vi "UHR-Fleezers Control (host) - 12.7.vi"() -> ()   [LabVIEW 2012] (continued)
              }
              frame True {
                n386 = stacked-sequence {
                  tunnel: w654 -> [_ _ _ _ _ _ _ _ _ w675 _ _]
                  tunnel: w653 -> [_ _ _ _ _ _ _ _ _ w673 _ _]
                  frame #0 {
                    n387 = property on="Save ave N" class="DigNum (strict)"("Val(Sgnl)"=1.0 ("Value (Signaling)")) -> ()  [unwired: 2 in, 2 out]
                  }
                  frame #1 {
                    n388 = Wait (ms)(milliseconds to wait=u32 500) -> ()  [unwired: 1 out]
                  }
                  frame #2 {
                    n389 = property on="Trap Delta (MHz)" class="DigNum (strict)"("Val(Sgnl)"="Offset 2 Start (MHz)") -> ()  [unwired: 2 in, 2 out]
                    n390 = Replace Array Subset(array=u32[] [0] ("Index Values"), new element="Offset 2 Set", index=0) -> (w659:u32[])
                    n391 = property on="Saved AOD Raster Scan Parameter Sets" class="Arr (strict)"("Index Values"=w659) -> ()  [unwired: 2 in, 2 out]
                  }
                  frame #3 {
                    n392 = Wait (ms)(milliseconds to wait=u32 500) -> ()  [unwired: 1 out]
                  }
                  frame #4 {
                    n393 = property on="Load parameters" class="Bool (strict)"("Val(Sgnl)"=TRUE ("Value (Signaling)")) -> ()  [unwired: 2 in, 2 out]
                  }
                  frame #5 {
                    n394 = Wait (ms)(milliseconds to wait=u32 500) -> ()  [unwired: 1 out]
                  }
                  frame #6 {
                    n395 = property on="Trap Raster Scan" class="Bool (strict)"("Val(Sgnl)"=TRUE ("Value (Signaling)")) -> ()  [unwired: 2 in, 2 out]
                  }
                  frame #7 {
                    n396 = Wait (ms)(milliseconds to wait=u32 2000) -> ()  [unwired: 1 out]
                  }
                  frame #8 {
                    n397 = while {
                      stop <- w668 stop-if-true
                      n398 = local read "Raster Scanning..."() -> (w671:bool)
                      n399 = local read "Saving..."() -> (w669:bool)
                      n400 = Wait (ms)(milliseconds to wait=u32 100) -> ()  [unwired: 1 out]
                      n401 = Not(x=w669) -> (.not. x?=w667:bool)
                      n402 = Not(x=w671) -> (.not. x?=w670:bool)
                      n403 = And(x=w670, y=w667) -> (x .and. y?=w668:bool)
                    }
                  }
                  frame #9 {
                    n404 = property on="Trap Delta (MHz)" class="DigNum (strict)"("Val(Sgnl)"=w675) -> ()  [unwired: 2 in, 2 out]
                    n405 = property on="Saved AOD Raster Scan Parameter Sets" class="Arr (strict)"("Index Values"=u32[] [0]) -> ()  [unwired: 2 in, 2 out]
                    n406 = property on="Save ave N" class="DigNum (strict)"("Val(Sgnl)"=w673) -> ()  [unwired: 2 in, 2 out]
                  }
                  frame #10 {
                    n407 = Wait (ms)(milliseconds to wait=u32 500) -> ()  [unwired: 1 out]
                  }
                  frame #11 {
                    n408 = property on="Load parameters" class="Bool (strict)"("Val(Sgnl)"=TRUE ("Value (Signaling)")) -> ()  [unwired: 2 in, 2 out]
                  }
                }
              }
            }
          }
          frame #9 {
            n409 = property on="Read Cal" class="Bool (strict)"("Val(Sgnl)"=TRUE ("Value (Signaling)")) -> ()  [unwired: 2 in, 2 out]
          }
          frame #10 {
            n410 = Wait (ms)(milliseconds to wait=u32 1000) -> ()  [unwired: 1 out]
          }
          frame #11 {
            n411 = property on="Fish for Tether" class="Bool (strict)"("Val(Sgnl)"=TRUE ("Value (Signaling)")) -> ()  [unwired: 2 in, 2 out]
          }
        }
        n412 = local write "Cal/Data Acq. Spot"(FALSE ("Cal/Data Acq. Spot")) -> ()
      }
      event "Dump Beads": Value Change {
        n413 = event-data() -> ()  [unwired: 1 in, 5 out]
        n414 = flat-sequence {
          tunnel: ["Dump spot flow on?"] -> w681
          tunnel: [w692] -> w682
          tunnel: w681 -> [w692]
          tunnel: w685 -> [w697]
          tunnel: w684 -> [w696]
          tunnel: [w694] -> w683
          tunnel: w682 -> [w694]
          tunnel: w683 -> [w707]
          frame #0 {
            w686 = FALSE ("Value (Signaling)")
            n415 = local read "Saving..."() -> (w688:bool)
            n416 = local write "Dump Beads"(FALSE ("Dump Beads")) -> ()
            n417 = property on="Inject Pump 3" class="Bool (strict)"("Val(Sgnl)"=w686) -> ()  [unwired: 2 in, 2 out]
            n418 = property on="Inject Pump 1" class="Bool (strict)"("Val(Sgnl)"=w686) -> ()  [unwired: 2 in, 2 out]
            n419 = local write "Stop Saving"(w688) -> ()
          }
          frame #1 {
            w689 = FALSE ("Fl. Triggered...")
            n420 = case shown="True" "Dump spot flow on?" {
              frame False {
              }
              frame True {
                n421 = property on="Sample Channel\nFlow" class="Bool (strict)"("Val(Sgnl)"=TRUE ("Stage Moving")) -> ()  [unwired: 2 in, 2 out]
              }
            }
            n422 = local write "Fl. Triggered..."(w689) -> ()
            n423 = local write "Tether"(w689) -> ()
            n424 = property on="Green Laser ON" class="Bool (strict)"("Val(Sgnl)"=w689) -> ()  [unwired: 2 in, 2 out]
            n425 = property on="Trap Pos. FB ON" class="Bool (strict)"("Val(Sgnl)"=w689) -> ()  [unwired: 2 in, 2 out]
            n426 = property on="Trap Trig. Fl." class="Bool (strict)"("Val(Sgnl)"=w689) -> ()  [unwired: 2 in, 2 out]
            n427 = property on="Fl. Triggered..." class="Bool (strict)"("Val(Sgnl)"=w689) -> ()  [unwired: 2 in, 2 out]
            n428 = property on="Dip for Protein" class="Bool (strict)"("Val(Sgnl)"=w689) -> ()  [unwired: 2 in, 2 out]
            n429 = property on="Pause dwell" class="Bool (strict)"("Val(Sgnl)"=w689) -> ()  [unwired: 2 in, 2 out]
          }
          frame #2 {
            n430 = property on="Trap Pos. FB Offset Factor" class="DigNum (strict)"("Val(Sgnl)"=i64 0 ("Value (Signaling)")) -> ()  [unwired: 2 in, 2 out]
          }
          frame #3 {
            n431 = local read "Saved Stage Positions"() -> (w698:dbl[][])
            n432 = local write "Stage Moving"(TRUE ("Stage Moving")) -> ()
            n433 = Array Subset(array=w698, index (row)=3 ("index"), length (row)=1 ("length"), index (col)=1 ("index"), length (col)=3 ("length")) -> (w703:dbl[][])
            n434 = Reshape Array(w703, 3 ("dimension size")) -> (w701:dbl[])
            n435 = Array To Cluster(array=w701) -> (cluster=w700:cluster{"[0]":dbl, "[1]":dbl, "[2]":dbl})
            n436 = call "Set Stage Position.vi"("Position"=w700, "error in"=w696, "VISA resource name in"=w697) -> ()  [unwired: 3 out]
          }
          frame #4 {
            w708 = FALSE ("Value (Signaling)")
            n437 = case shown="True" w707 {
              frame False {
              }
              frame True {
                n438 = property on="Sample Channel\nFlow" class="Bool (strict)"("Val(Sgnl)"=FALSE ("Stage Moving")) -> ()  [unwired: 2 in, 2 out]
              }
            }
            n439 = property on="Trap 1 (ON/OFF)" class="Bool (strict)"("Val(Sgnl)"=w708) -> ()  [unwired: 2 in, 2 out]
            n440 = property on="Trap 2 (ON/OFF)" class="Bool (strict)"("Val(Sgnl)"=w708) -> ()  [unwired: 2 in, 2 out]
            n441 = call <vilib>:"Beep.vi"() -> ()  [unwired: 3 in, 9 out]
          }
          frame #5 {
            n442 = property on="Move Cap. 2 (ADig Top)" class="Bool (strict)"("Val(Sgnl)"=TRUE ("Value (Signaling)")) -> ()  [unwired: 2 in, 2 out]
            n443 = property on="Tab Control" class="TabCtl (strict)"("Val(Sgnl)"=T26."Status" ("Value (Signaling)")) -> ()  [unwired: 2 in, 2 out]
          }
        }
      }
      event "Dip for Protein": Value Change {
        n444 = event-data() -> ()  [unwired: 1 in, 5 out]
        n445 = case shown="True" "Dip for Protein" {
          tunnel: w714 -> [_ w716]
          tunnel: w713 -> [_ w715]
          frame False {
          }
          frame True {
            n446 = while {
              tunnel: w716 -> [w727]
              tunnel: w715 -> [w726]
              i -> [w721]
              stop <- w723 stop-if-true
              n447 = Increment(x=w721) -> (x+1=→"Dip #":i32)
              n448 = flat-sequence {
                tunnel: w726 -> [w738]
                tunnel: w727 -> [w739]
                tunnel: [w739] -> w731
                tunnel: [w738] -> w730
                tunnel: [w732] -> w717
                tunnel: [w744] -> w725
                tunnel: [w745] -> w724
                tunnel: w731 -> [w746]
                tunnel: w730 -> [w747]
                tunnel: [w742] -> w718
                tunnel: w717 -> [w742]
                tunnel: [w755] -> w729
                tunnel: w725 -> [w755]
                tunnel: [w754] -> w728
                tunnel: w724 -> [w754]
                tunnel: [w751] -> w722
                tunnel: [w750] -> w719
                tunnel: w718 -> [w750]
                tunnel: w728 -> [w775]
                tunnel: w729 -> [w776]
                tunnel: w722 -> [w777]
                tunnel: w719 -> [w774]
                tunnel: [w833] -> w723
                frame #0 {
                  n449 = local read "Trap Pos. FB ON"() -> (w732:bool)
                  n450 = Compound Arithmetic op=AND("Flow ON\nduring dip?", "FB OFF when \nflow ON", w732) -> (w733:bool)
                  n451 = case shown="True" "Move trap \nbefore dip move?" {
                    frame False {
                    }
                    frame True {
                      n452 = property on="Trap Delta (MHz)" class="DigNum (strict)"("Val(Sgnl)"="Dipping Delta (MHz)") -> ()  [unwired: 2 in, 2 out]
                    }
                  }
                  n453 = property on="Green Laser ON" class="Bool (strict)"("Val(Sgnl)"="Green ON\nbefore dip?") -> ()  [unwired: 2 in, 2 out]
                  n454 = property on="Sample Channel\nFlow" class="Bool (strict)"("Val(Sgnl)"="Flow ON\nduring dip?") -> ()  [unwired: 2 in, 2 out]
                  n455 = case shown="True" w733 {
                    frame False {
                    }
                    frame True {
                      n456 = property on="Trap Pos. FB ON" class="Bool (strict)"("Val(Sgnl)"=FALSE ("Value (Signaling)")) -> ()  [unwired: 2 in, 2 out]
                    }
                  }
                }
                frame #1 {
                  n457 = local read "Saved Stage Positions"() -> (w749:dbl[][])
                  n458 = local write "Cancel dwell"(FALSE ("Cancel dwell")) -> ()
                  n459 = call "move to saved stage position.vi"("error in"=w747, "Stage VISA resource name in"=w746, "Position"="Dip Stage \nPosition", "Saved Stage Positions"=w749) -> ("VISA resource name out"=w744:refnum<visa-resource-name>, "error out"=w745:errorcluster)
                }
                frame #2 {
                  n460 = node-c288() -> (w753:T23)  [unwired: 4 in]
                  n461 = timed-loop {
                    timing: w753 -> [_]
                    timing-out: [_] -> w752
                    tunnel: [w759] -> w751
                    i -> [w756]
                    stop <- w760 stop-if-true
                    n462 = node-c288() -> ()  [unwired: 1 in, 1 out]
                    n463 = Greater Or Equal?(x=w756, y="Dip Duration (s)") -> (x >= y?=w768:bool)
                    n464 = local read "Dip for Protein"() -> (w761:bool)
                    n465 = local read "Dump Beads"() -> (w758:bool)
                    n466 = local read "Cancel dwell"() -> (w767:bool)
                    n467 = local read "Pause dwell"() -> (w764:bool)
                    n468 = Not(x=w761) -> (.not. x?=w766:bool)
                    n469 = Compound Arithmetic op=OR(w767, w768, w766) -> (w765:bool)
                    n470 = Select(t=FALSE, s=w764, f=w765) -> (s? t:f=w762:bool)
                    n471 = Not(x=w758) -> (.not. x?=w757:bool)
                    n472 = node-c288() -> ()  [unwired: 1 in, 1 out]
                    n473 = And(x=w761, y=w757) -> (x .and. y?=w759:bool)
                    n474 = Or(x=w762, y=w758) -> (x .or. y?=w760:bool)
                    "Dip Time (s)" <- w756
                  }
                  n475 = node-c288(w752) -> ()  [unwired: 1 out]
                }
                frame #3 {
                  n476 = case shown="True" w777 {
                    tunnel: w776 -> [_ w782]
                    tunnel: w775 -> [_ w781]
                    tunnel: w774 -> [_ w778]
                    frame False {
                    }
                    frame True {
                      n477 = flat-sequence {
                        tunnel: w781 -> [w786]
                        tunnel: w782 -> [w787]
                        tunnel: [w787] -> w780
                        tunnel: [w786] -> w779
                        tunnel: w778 -> [w783]
                        tunnel: w780 -> [w797]
                        tunnel: w779 -> [w796]
                        tunnel: w778 -> [w805]
                        frame #0 {
                          n478 = local read "Sample Channel\nFlow"() -> (w785:bool)
                          n479 = case shown="True" w785 {
                            tunnel: "Flow ON \nduring return\nfrom dip?" -> [w788 w791]
                            tunnel: w783 -> [_ w790]
                            frame False {
                              n480 = case shown="True" w788 {
                                frame False {
                                }
                                frame True {
                                n481 = property on="Sample Channel\nFlow" class="Bool (strict)"("Val(Sgnl)"=TRUE ("Value (Signaling)")) -> ()  [unwired: 2 in, 2 out]
                                }
                              }
                            }
                            frame True {
                              n482 = case shown="False" w791 {
                                tunnel: w790 -> [w792 _]
                                frame False {
                                n483 = property on="Trap Pos. FB ON" class="Bool (strict)"("Val(Sgnl)"=w792) -> ()  [unwired: 2 in, 2 out]
                                n484 = property on="Sample Channel\nFlow" class="Bool (strict)"("Val(Sgnl)"=FALSE ("Value (Signaling)")) -> ()  [unwired: 2 in, 2 out]
                                }
                                frame True {
                                }
                              }
                            }
                          }
                        }
                        frame #1 {
                          # "For turning on green laser before stage reaches lower spot"
                          n485 = case shown="True" "Green ON\nafter start\nreturn?" {
                            frame False {
                            }
                            frame True {
                              n486 = flat-sequence {
                                frame #0 {
                                n487 = Multiply(x="Green delay after \nstart return (s)", y=1000.0) -> (x*y=w802:dbl)
                                n488 = Wait (ms)(milliseconds to wait=w802) -> ()  [unwired: 1 out]
                                }
                                frame #1 {
                                n489 = property on="Green Laser ON" class="Bool (strict)"("Val(Sgnl)"=TRUE ("Value (Signaling)")) -> ()  [unwired: 2 in, 2 out]
                                }
                              }
                            }
                          }
                          n490 = local read "Saved Stage Positions"() -> (w800:dbl[][])
                          n491 = local write "Cancel dwell"(FALSE ("Cancel dwell")) -> ()
                          n492 = call "move to saved stage position.vi"("error in"=w796, "Stage VISA resource name in"=w797, "Position"="Return Stage \nPosition", "Saved Stage Positions"=w800) -> ("error out"=w798:errorcluster)  [unwired: 1 out]
                          n493 = local write "Stage Control Serial Error"(w798) -> ()
                        }
                        frame #2 {
                          n494 = property on="Trap Pos. FB ON" class="Bool (strict)"("Val(Sgnl)"=w805) -> ()  [unwired: 2 in, 2 out]
                          n495 = case shown="True" "Green ON \nafter return?" {
                            frame False {
                            }
                            frame True {
                              n496 = property on="Green Laser ON" class="Bool (strict)"("Val(Sgnl)"=TRUE ("Value (Signaling)")) -> ()  [unwired: 2 in, 2 out]
                            }
                          }
                          n497 = case shown="True" "Move trap after return?" {
                            frame False {
                            }
                            frame True {
                              n498 = property on="Trap Delta (MHz)" class="DigNum (strict)"("Val(Sgnl)"="Dip Trap Delta 2 (MHz)") -> ()  [unwired: 2 in, 2 out]
                            }
                          }
                          n499 = case shown="True" "Save data after return?" {
                            frame False {
                            }
                            frame True {
                              n500 = property on="Start Saving" class="Bool (strict)"("Val(Sgnl)"=TRUE ("Value (Signaling)")) -> ()  [unwired: 2 in, 2 out]
                            }
                          }
                          n501 = property on="Sample Channel\nFlow" class="Bool (strict)"("Val(Sgnl)"="Flow ON\nduring daq?") -> ()  [unwired: 2 in, 2 out]
                        }
                        frame #3 {
                          n502 = node-c288() -> (w814:T23)  [unwired: 4 in]
                          n503 = timed-loop {
                            timing: w814 -> [_]
                            timing-out: [_] -> w813
                            i -> [w815]
                            stop <- w817 stop-if-true
                            n504 = node-c288() -> ()  [unwired: 1 in, 1 out]
                            n505 = local read "Dump Beads"() -> (w816:bool)
                            n506 = Greater Or Equal?(x=w815, y="Dwell Duration (s)") -> (x >= y?=w822:bool)
                            n507 = local read "Dip for Protein"() -> (w819:bool)
                            n508 = Not(x=w819) -> (.not. x?=w818:bool)
                            n509 = Compound Arithmetic op=OR(w822, "Cancel dwell", w818) -> (w821:bool)
                            n510 = node-c288() -> ()  [unwired: 1 in, 1 out]
                            n511 = Select(t=FALSE, s="Pause dwell", f=w821) -> (s? t:f=w824:bool)
                            n512 = Or(x=w824, y=w816) -> (x .or. y?=w817:bool)
                            "Dwell Time (s)" <- w815
                          }
                          n513 = node-c288(w813) -> ()  [unwired: 1 out]
                        }
                      }
                    }
                  }
                }
                frame #4 {
                  n514 = local read "Dip for Protein"() -> (w834:bool)
                  n515 = local read "Dump Beads"() -> (w831:bool)
                  n516 = local write "Cancel dwell"(FALSE ("Cancel dwell")) -> ()
                  n517 = Not(x=w834) -> (.not. x?=w835:bool)
                  n518 = Not(x="Cont. Repeat Dipping?") -> (.not. x?=w837:bool)
                  n519 = Compound Arithmetic op=OR(w835, w837, w831) -> (w833:bool)
                }
              }
            }
          }
        }
      }
      event "Profile": Value Change {
        n520 = event-data() -> ()  [unwired: 1 in, 5 out]
        n521 = flat-sequence {
          tunnel: w846 -> [w849]
          tunnel: w845 -> [w857]
          tunnel: [w851] -> w844
          tunnel: [w850] -> w843
          tunnel: [w848] -> w841
          tunnel: [w847] -> w838
          tunnel: w844 -> [w864]
          tunnel: w843 -> [w863]
          tunnel: [w861] -> w842
          tunnel: w841 -> [w862]
          tunnel: [w860] -> w840
          tunnel: [w859] -> w839
          tunnel: w838 -> [w859]
          tunnel: w842 -> [w868]
          tunnel: w840 -> [w867]
          tunnel: w839 -> [w866]
          frame #0 {
            n522 = call "Read Stage Position.vi"("error in"=w857, "VISA resource name in"=w849) -> ("Current Position"=w847:cluster{dbl, dbl, dbl}, "error out"=w850:errorcluster, "VISA resource name out"=w848:refnum<visa-resource-name>)  [unwired: 1 out]
            "Current Position" <- w847
            n523 = local write "Stage Control Serial Error"(w850) -> ()
            n524 = Unbundle(w847) -> (w854:dbl, w856:dbl, w852:dbl)
            n525 = Add(x=w856, y="Y change (mm)") -> (x+y=w853:dbl)
            n526 = Bundle(w854, w853, w852) -> (w851:cluster{dbl, dbl, dbl})  [unwired: 1 in]
          }
          frame #1 {
            # "move to new position and start saving"
            n527 = local write "Stage Moving"(TRUE ("Stage Moving")) -> ()
            n528 = local write "Start Saving"(TRUE ("Start Saving")) -> ()
            n529 = call "Set Stage Position.vi"("Position"=w864, "error in"=w863, "VISA resource name in"=w862) -> ("error out"=w860:errorcluster, "VISA resource name out"=w861:refnum<visa-resource-name>)  [unwired: 1 out]
          }
          frame #2 {
            # "go back to start"
            n530 = call "Set Stage Position.vi"("Position"=w866, "error in"=w867, "VISA resource name in"=w868) -> ()  [unwired: 3 out]
          }
          frame #3 {
            # "stop saving"
            n531 = local write "Stop Saving"(TRUE ("Stop Saving")) -> ()
            n532 = local write "Stage Moving"(FALSE ("Stage Moving")) -> ()
          }
        }
      }
      event "Move to Position 1", "Move to Position 2", "Move to Position 3", "Move to Position 4", "Move to Position 5", "Lower Ch. Cap.": Value Change {
        n533 = event-data() -> ()  [unwired: 1 in, 5 out]
        n534 = Or(x="Move to Position 5", y="Lower Ch. Cap.") -> (x .or. y?=w874:bool)
        n535 = Build Array("Move to Position 1", "Move to Position 2", "Move to Position 3", "Move to Position 4", w874) -> (w877:bool[])
        n536 = Boolean Array To Number(Boolean array=w877) -> (number=w876:u32)
        n537 = Logarithm Base 2(1:w876) -> (0:w875:dbl)
        n538 = flat-sequence {
          tunnel: w875 -> [w886]
          tunnel: w872 -> [w884]
          tunnel: w871 -> [w883]
          frame #0 {
            n539 = local read "Saved Stage Positions"() -> (w894:dbl[][])
            n540 = Array Subset(array=w894, index (row)=w886, length (row)=1 ("length"), index (col)=1 ("index"), length (col)=3 ("length")) -> (w891:dbl[][])
            n541 = Reshape Array(w891, 3 ("dimension size")) -> (w889:dbl[])
            n542 = Array To Cluster(array=w889) -> (cluster=w888:cluster{"[0]":dbl, "[1]":dbl, "[2]":dbl})
            n543 = call "Set Stage Position.vi"("Position"=w888, "error in"=w883, "VISA resource name in"=w884) -> ("error out"=w887:errorcluster)  [unwired: 2 out]
            n544 = local write "Stage Moving"(TRUE ("Stage Moving")) -> ()
            n545 = local write "Stage Control Serial Error"(w887) -> ()
          }
          frame #1 {
            n546 = local write "Stage Moving"(FALSE ("Stage Moving")) -> ()
            n547 = call <vilib>:"Beep.vi"() -> ()  [unwired: 3 in, 9 out]
          }
        }
      }
      event "Got ADig bead": Value Change {
        n548 = event-data() -> ()  [unwired: 1 in, 5 out]
        n549 = flat-sequence {
          frame #0 {
            n550 = local read "Cap 1 Samp Flow ON"() -> (w898:bool)
            n551 = case shown="True" w898 {
              frame False {
              }
              frame True {
                n552 = property on="Sample Channel\nFlow" class="Bool (strict)"("Val(Sgnl)"=TRUE ("Value (Signaling)")) -> ()  [unwired: 2 in, 2 out]
              }
            }
          }
          frame #1 {
            n553 = property on="Inject Pump 3" class="Bool (strict)"("Val(Sgnl)"=FALSE ("Value (Signaling)")) -> ()  [unwired: 2 in, 2 out]
          }
          frame #2 {
            n554 = property on="Move Cap. 1 (DNA Bottom)" class="Bool (strict)"("Val(Sgnl)"=TRUE ("Value (Signaling)")) -> ()  [unwired: 2 in, 2 out]
          }
        }
      }
      event "Force FB Data\nScript": Value Change {
        n555 = event-data() -> ()  [unwired: 1 in, 5 out]
        n556 = flat-sequence {
          tunnel: w907 -> [w911]
          tunnel: w908 -> [w912]
          tunnel: [w912] -> w903
          tunnel: [w911] -> w902
          tunnel: w903 -> [w915]
          tunnel: w902 -> [w914]
          tunnel: ["Trap Trig Fl."] -> w904
          tunnel: [w940] -> w905
          tunnel: w904 -> [w940]
          tunnel: [w944] -> w906
          tunnel: w905 -> [w944]
          tunnel: w906 -> [w946]
          frame #0 {
            n557 = property on="Trap Delta (MHz)" class="DigNum (strict)"("Val(Sgnl)"="Trap Delta Before Moving") -> ()  [unwired: 2 in, 2 out]
          }
          frame #1 {
            n558 = local read "Saved Stage Positions"() -> (w917:dbl[][])
            n559 = local write "FB Trap Pos Offset"(0.0 ("FB Trap Pos Offset")) -> ()
            n560 = property on="Trap Pos. FB Offset Factor" class="DigNum (strict)"("Val(Sgnl)"=i64 0 ("Value (Signaling)")) -> ()  [unwired: 2 in, 2 out]
            n561 = local write "Stage Moving"(TRUE ("Stage Moving")) -> ()
            n562 = call "move to saved stage position.vi"("error in"=w914, "Stage VISA resource name in"=w915, "Position"="Stage Position To Establish FB", "Saved Stage Positions"=w917) -> ("error out"=w913:errorcluster)  [unwired: 1 out]
            n563 = local write "Stage Control Serial Error"(w913) -> ()
          }
          frame #2 {
            n564 = call <vilib>:"Beep.vi"() -> ()  [unwired: 3 in, 9 out]
            n565 = Multiply(x="Wait (s)", y=u32 1000 ("milliseconds to wait")) -> (x*y=w924:u32)
            n566 = property on="Trap Delta (MHz)" class="DigNum (strict)"("Val(Sgnl)"="Starting \nTrap Delta (MHz)") -> ()  [unwired: 2 in, 2 out]
            n567 = local write "Stage Moving"(FALSE ("Stage Moving")) -> ()
            n568 = Wait (ms)(milliseconds to wait=w924) -> ()  [unwired: 1 out]
            n569 = property on="Tab Control 2" class="TabCtl (strict)"("Val(Sgnl)"=T6."Feedback on Trap Position" ("Value (Signaling)")) -> ()  [unwired: 2 in, 2 out]
            n570 = property on="Tab Control" class="TabCtl (strict)"("Val(Sgnl)"=T27."Trap Control (RF)" ("Value (Signaling)")) -> ()  [unwired: 2 in, 2 out]
          }
          frame #3 {
            n571 = property on="Set Reading to\nSetpoint" class="Bool (strict)"("Val(Sgnl)"=TRUE ("Value (Signaling)")) -> ()  [unwired: 2 in, 2 out]
            n572 = Wait (ms)(milliseconds to wait=u32 500) -> ()  [unwired: 1 out]
          }
          frame #4 {
            n573 = property on="Trap Pos. FB ON" class="Bool (strict)"("Val(Sgnl)"=TRUE ("Value (Signaling)")) -> ()  [unwired: 2 in, 2 out]
            n574 = Wait (ms)(milliseconds to wait=u32 250) -> ()  [unwired: 1 out]
          }
          frame #5 {
            n575 = case shown="False" "Trap Trig Fl." {
              frame False {
                n576 = case shown="True" "Green ON after FB ON?" {
                  selector: "Green ON after FB ON?" -> [_ w939]
                  frame False {
                  }
                  frame True {
                    n577 = property on="Green Laser ON" class="Bool (strict)"("Val(Sgnl)"=w939) -> ()  [unwired: 2 in, 2 out]
                  }
                }
              }
              frame True {
              }
            }
            n578 = case shown="True" "Remove Action Offset" {
              tunnel: TRUE ("Value (Signaling)") -> [w936 w937]
              frame False {
                n579 = property on="Remove Unwinding Offset" class="Bool (strict)"("Val(Sgnl)"=w936) -> ()  [unwired: 2 in, 2 out]
              }
              frame True {
                n580 = property on="Remove Action Offset" class="Bool (strict)"("Val(Sgnl)"=w937) -> ()  [unwired: 2 in, 2 out]
              }
            }
            n581 = Wait (ms)(milliseconds to wait=u32 250) -> ()  [unwired: 1 out]
          }
          frame #6 {
            n582 = property on="Start Saving" class="Bool (strict)"("Val(Sgnl)"=TRUE ("Value (Signaling)")) -> ()  [unwired: 2 in, 2 out]
            n583 = Wait (ms)(milliseconds to wait=u32 5000) -> ()  [unwired: 1 out]
          }
          frame #7 {
            w943 = TRUE ("Value (Signaling)")
            n584 = property on="Rem fb disp offset" class="Bool (strict)"("Val(Sgnl)"=w943) -> ()  [unwired: 2 in, 2 out]
            n585 = property on="Remove Offset" class="Bool (strict)"("Val(Sgnl)"=w943) -> ()  [unwired: 2 in, 2 out]
            n586 = Wait (ms)(milliseconds to wait=u32 100) -> ()  [unwired: 1 out]
          }
          frame #8 {
            n587 = case shown="True" w946 {
              frame False {
              }
              frame True {
                n588 = local write "Trap Trig. Fl."(TRUE ("Value (Signaling)")) -> ()
              }
            }
          }
          frame #9 {
            n589 = case shown="True" "Start dipping after?" {
              frame False {
              }
              frame True {
                n590 = flat-sequence {
                  frame #0 {
                    n591 = Multiply(x="Delay before dipping (s)", y=1000.0) -> (x*y=w950:dbl)
                    n592 = Wait (ms)(milliseconds to wait=w950) -> ()  [unwired: 1 out]
                  }
                  frame #1 {
                    n593 = property on="Dip for Protein" class="Bool (strict)"("Val(Sgnl)"=TRUE ("Value (Signaling)")) -> ()  [unwired: 2 in, 2 out]
                    n594 = local write "Scripts"(T1."Dipping" ("Scripts")) -> ()
                  }
                }
              }
            }
          }
        }
      }
      event "Fixed Traps Data\nScript": Value Change {
        n595 = event-data() -> ()  [unwired: 1 in, 5 out]
        n596 = flat-sequence {
          frame #0 {
            n597 = case shown="True" "Green ON" {
              frame False {
              }
              frame True {
                n598 = property on="Green Laser ON" class="Bool (strict)"("Val(Sgnl)"=TRUE) -> ()  [unwired: 2 in, 2 out]
              }
            }
            n599 = local write "Offset (nm)"(0.0 ("Offset (nm)")) -> ()
            n600 = property on="Sample Channel\nFlow" class="Bool (strict)"("Val(Sgnl)"=FALSE ("Value (Signaling)")) -> ()  [unwired: 2 in, 2 out]
            n601 = property on="Trap Delta (MHz)" class="DigNum (strict)"("Val(Sgnl)"="Fixed Traps Trap Delta (MHz)") -> ()  [unwired: 2 in, 2 out]
          }
          frame #1 {
            n602 = Wait (ms)(milliseconds to wait=u32 1000) -> ()  [unwired: 1 out]
          }
          frame #2 {
            n603 = local write "Start Saving"(TRUE ("Start Saving")) -> ()
          }
          frame #3 {
            n604 = local read "Bead Sep. Int. Time (s)"() -> (w961:dbl)
            n605 = Multiply(x=w961, y=1000.0) -> (x*y=w963:dbl)
            n606 = Wait (ms)(milliseconds to wait=w963) -> ()  [unwired: 1 out]
          }
          frame #4 {
            n607 = property on="Remove Offset" class="Bool (strict)"("Val(Sgnl)"=TRUE ("Value (Signaling)")) -> ()  [unwired: 2 in, 2 out]
          }
          frame #5 {
            n608 = property on="Dip for Protein" class="Bool (strict)"("Val(Sgnl)"="Start dipping after?") -> ()  [unwired: 2 in, 2 out]
          }
        }
      }
      event "Got DNA bead": Value Change {
        n609 = event-data() -> ()  [unwired: 1 in, 5 out]
        n610 = flat-sequence {
          frame #0 {
            n611 = local read "Daq spot flow on"() -> (w968:bool)
            n612 = case shown="True" w968 {
              frame False {
              }
              frame True {
                n613 = property on="Sample Channel\nFlow" class="Bool (strict)"("Val(Sgnl)"=TRUE ("Value (Signaling)")) -> ()  [unwired: 2 in, 2 out]
              }
            }
            n614 = property on="Got DNA bead" class="Bool"("Key Focus"=FALSE) -> ()  [unwired: 2 in, 2 out]
          }
          frame #1 {
            n615 = property on="Inject Pump 1" class="Bool (strict)"("Val(Sgnl)"=FALSE ("Value (Signaling)")) -> ()  [unwired: 2 in, 2 out]
          }
          frame #2 {
            n616 = property on="Cal/Data Acq. Spot" class="Bool (strict)"("Val(Sgnl)"=TRUE ("Value (Signaling)")) -> ()  [unwired: 2 in, 2 out]
          }
        }
      }
      event "Take Stepping Data": Value Change {
        n617 = event-data() -> ()  [unwired: 1 in, 5 out]
        n618 = local read "Save ave N"() -> (w980:dbl)
        n619 = flat-sequence {
          tunnel: w980 -> [w982]
          tunnel: [w982] -> w975
          tunnel: [w984] -> w976
          tunnel: w975 -> [w984]
          tunnel: [w986] -> w977
          tunnel: w976 -> [w986]
          tunnel: [w989] -> w978
          tunnel: w977 -> [w989]
          tunnel: [w991] -> w979
          tunnel: w978 -> [w991]
          tunnel: [w993] -> w973
          tunnel: w979 -> [w993]
          tunnel: w973 -> [w996]
          tunnel: [w996] -> w972
          tunnel: w972 -> [w997]
          tunnel: [w997] -> w974
          tunnel: w974 -> [w1003]
          frame #0 {
            n620 = property on="Save ave N" class="DigNum (strict)"("Val(Sgnl)"="Save ave factor") -> ()  [unwired: 2 in, 2 out]
          }
          frame #1 {
            n621 = Wait (ms)(milliseconds to wait=u32 100) -> ()  [unwired: 1 out]
          }
          frame #2 {
            n622 = local read "Offset 2 Start (MHz)"() -> (w988:dbl)
            n623 = property on="Saved AOD Raster Scan Parameter Sets" class="Arr (strict)"("Index Values"=u32[] [2]) -> ()  [unwired: 2 in, 2 out]
            n624 = property on="Trap Delta (MHz)" class="DigNum (strict)"("Val(Sgnl)"=w988) -> ()  [unwired: 2 in, 2 out]
          }
          frame #3 {
            n625 = property on="Load parameters" class="Bool (strict)"("Val(Sgnl)"=TRUE ("Value (Signaling)")) -> ()  [unwired: 2 in, 2 out]
          }
          frame #4 {
            n626 = Wait (ms)(milliseconds to wait=u32 100) -> ()  [unwired: 1 out]
          }
          frame #5 {
            n627 = property on="Trap Raster Scan" class="Bool (strict)"("Val(Sgnl)"=TRUE ("Value (Signaling)")) -> ()  [unwired: 2 in, 2 out]
          }
          frame #6 {
            n628 = Wait (ms)(milliseconds to wait=u32 1000) -> ()  [unwired: 1 out]
          }
          frame #7 {
            n629 = while {
              stop <- w1000 stop-if-true
              n630 = local read "Raster Scanning..."() -> (w1002:bool)
              n631 = local read "Saving..."() -> (w1001:bool)
              n632 = Not(x=w1001) -> (.not. x?=w998:bool)
              n633 = Not(x=w1002) -> (.not. x?=w999:bool)
              n634 = And(x=w999, y=w998) -> (x .and. y?=w1000:bool)
            }
          }
          frame #8 {
            n635 = property on="Save ave N" class="DigNum (strict)"("Val(Sgnl)"=w1003) -> ()  [unwired: 2 in, 2 out]
          }
        }
      }
      event "Step Size (nm)": Value Change {
        n636 = event-data() -> ()  [unwired: 1 in, 5 out]
        n637 = flat-sequence {
          frame #0 {
            n638 = property on="Saved AOD Raster Scan Parameter Sets" class="Arr (strict)"("Index Values"=u32[] [1]) -> ()  [unwired: 2 in, 2 out]
          }
          frame #1 {
            n639 = Multiply(x="N Steps", y="Step Size (nm)") -> (x*y=w1005:dbl)
            n640 = property on="Scan Speed AOD (nm/s) 2" class="DigNum (strict)"("Value"="Step Size (nm)") -> ()  [unwired: 2 in, 2 out]
            n641 = property on="Step Size AOD (nm) 2" class="DigNum (strict)"("Value"="Step Size (nm)") -> ()  [unwired: 2 in, 2 out]
            n642 = property on="Scan Range AOD (nm) 2" class="DigNum (strict)"("Value"=w1005) -> ()  [unwired: 2 in, 2 out]
          }
        }
      }
      event "Take Detection Laser\nImage": Value Change {
        n643 = event-data() -> ()  [unwired: 1 in, 5 out]
        n644 = flat-sequence {
          tunnel: [w1033] -> w1023
          tunnel: [w1032] -> w1016
          tunnel: [w1031] -> w1008
          tunnel: [w1036] -> w1024
          tunnel: w1023 -> [w1036]
          tunnel: [w1035] -> w1017
          tunnel: w1016 -> [w1035]
          tunnel: [w1034] -> w1009
          tunnel: w1008 -> [w1034]
          tunnel: [w1040] -> w1025
          tunnel: w1024 -> [w1040]
          tunnel: [w1039] -> w1018
          tunnel: w1017 -> [w1039]
          tunnel: [w1038] -> w1010
          tunnel: w1009 -> [w1038]
          tunnel: [w1046] -> w1026
          tunnel: w1025 -> [w1046]
          tunnel: [w1045] -> w1019
          tunnel: w1018 -> [w1045]
          tunnel: [w1044] -> w1011
          tunnel: w1010 -> [w1044]
          tunnel: [w1050] -> w1027
          tunnel: w1026 -> [w1050]
          tunnel: [w1049] -> w1020
          tunnel: w1019 -> [w1049]
          tunnel: [w1048] -> w1012
          tunnel: w1011 -> [w1048]
          tunnel: [w1054] -> w1028
          tunnel: w1027 -> [w1054]
          tunnel: [w1053] -> w1021
          tunnel: w1020 -> [w1053]
          tunnel: [w1052] -> w1013
          tunnel: w1012 -> [w1052]
          tunnel: [w1058] -> w1029
          tunnel: w1028 -> [w1058]
          tunnel: [w1057] -> w1022
          tunnel: w1021 -> [w1057]
          tunnel: [w1056] -> w1014
          tunnel: w1013 -> [w1056]
          tunnel: w1029 -> [w1064]
          tunnel: w1022 -> [w1063]
          tunnel: [w1061] -> w1015
          tunnel: w1014 -> [w1061]
          tunnel: w1015 -> [w1065]
          frame #0 {
            n645 = local read "Laser interlacing mode"() -> (w1032:enum32{"Laser ON", "Laser OFF", "Interlace"})
            n646 = local read "Green FB On/Off"() -> (w1031:bool)
            n647 = local read "Green Laser ON"() -> (w1033:bool)
          }
          frame #1 {
            n648 = property on="Green FB On/Off" class="Bool (strict)"("Val(Sgnl)"=FALSE ("Value (Signaling)")) -> ()  [unwired: 2 in, 2 out]
          }
          frame #2 {
            n649 = property on="Green Laser ON" class="Bool (strict)"("Val(Sgnl)"=TRUE ("Value (Signaling)")) -> ()  [unwired: 2 in, 2 out]
            n650 = property on="Flip Green Filter" class="Bool (strict)"("Val(Sgnl)"=TRUE ("Value (Signaling)")) -> ()  [unwired: 2 in, 2 out]
            n651 = property on="Laser interlacing mode" class="RadioBtnsControl (strict)"("Val(Sgnl)"=enum32{"Laser ON", "Laser OFF", "Interlace"}."Laser ON" ("Value (Signaling)")) -> ()  [unwired: 2 in, 2 out]
          }
          frame #3 {
            n652 = Wait (ms)(milliseconds to wait=u32 500) -> ()  [unwired: 1 out]
          }
          frame #4 {
            n653 = property on="Confocal Image" class="Bool (strict)"("Val(Sgnl)"=TRUE ("Value (Signaling)")) -> ()  [unwired: 2 in, 2 out]
          }
          frame #5 {
            n654 = Wait (ms)(milliseconds to wait=u32 2000) -> ()  [unwired: 1 out]
          }
          frame #6 {
            n655 = while {
              stop <- w1059 stop-if-true
              n656 = local read "Saving..."() -> (w1060:bool)
              n657 = Not(x=w1060) -> (.not. x?=w1059:bool)
            }
          }
          frame #7 {
            n658 = property on="Flip Green Filter" class="Bool (strict)"("Val(Sgnl)"=TRUE ("Value (Signaling)")) -> ()  [unwired: 2 in, 2 out]
            n659 = property on="Green Laser ON" class="Bool (strict)"("Val(Sgnl)"=w1064) -> ()  [unwired: 2 in, 2 out]
            n660 = property on="Laser interlacing mode" class="RadioBtnsControl (strict)"("Val(Sgnl)"=w1063) -> ()  [unwired: 2 in, 2 out]
          }
          frame #8 {
            n661 = property on="Green FB On/Off" class="Bool (strict)"("Val(Sgnl)"=w1065) -> ()  [unwired: 2 in, 2 out]
          }
        }
      }
      event "Stop All": Value Change {
        # "Stopping blue laser before shutting off program"
        n662 = event-data() -> ()  [unwired: 1 in, 5 out]
        n663 = local read "Delay (ms)"() -> (w1068:i32)
        n664 = call "serial write macro.vi"("String"="l0", "Delay (ms)"=w1068, "VISA resource name"=w1071) -> ("read buffer"=w1066:string, "error out"=w1067:errorcluster, "VISA resource name out"=w1070:refnum<visa-resource-name>)
        n665 = local write "read blue buffer"(w1066) -> ()
        n666 = local write "Blue Error Out"(w1067) -> ()
        n667 = VISA Close(VISA resource name=w1070) -> ()  [unwired: 1 in, 1 out]
        n668 = local read "Stop All"() -> (w1072:bool)
      }
    }
    n669 = node-c288() -> ()  [unwired: 1 in, 1 out]
  }
  n670 = node-c288() -> (w12:T23)  [unwired: 4 out]
  n671 = timed-loop "Oscillate Trap/AOM (fishing, conjugate plane alignment)" {
    tunnel: w18 -> [w1074]
    tunnel: [w1073] -> w131
    timing: w126 -> [_]
    timing-out: [_] -> w125
    stop <- w1073 stop-if-true
    n672 = node-c288() -> ()  [unwired: 2 out]
    n673 = event shown="[0] \"Oscillate Set 1\", \"Fish for Tether\": Value Change" {
      selector: _ -> [_ _ _]
      dyn-events: _ -> [_ _ _]
      timeout: _ -> [_ _ _]
      tunnel: w1074 -> [w1081 _ _]
      tunnel: [FALSE ("Stop All") _ w1679] -> w1073
      event "Oscillate Set 1", "Fish for Tether": Value Change {
        n674 = event-data() -> ()  [unwired: 6 out]
        n675 = local read "Oscillate Set 1"() -> (w1080:bool)
        n676 = Or(x=w1080, y="Fish for Tether") -> (x .or. y?=w1078:bool)
        n677 = case shown="True" w1078 {
          tunnel: w1081 -> [_ w1084]
          tunnel: "Fish for Tether" -> [_ w1083]
          frame False {
          }
          frame True {
            n678 = case shown="True" w1083 {
              selector: w1083 -> [w1087 w1093]
              tunnel: [w1087 w1093] -> w1082
              frame False {
              }
              frame True {
                n679 = local write "Scan axis 2"(TRUE) -> ()
                n680 = local write "Tether"(FALSE ("Tether")) -> ()
                n681 = local read "Flow ON during cal?"() -> (w1088:bool)
                n682 = property on="Trap Delta (MHz)" class="DigNum (strict)"("Val(Sgnl)"="Furthest Delta (MHz)") -> ()  [unwired: 2 in, 2 out]
                n683 = Or(x="Flow ON during \nfishing?", y=w1088) -> (x .or. y?=w1089:bool)
                n684 = Wait (ms)(milliseconds to wait=u32 500) -> ()  [unwired: 1 out]
                n685 = property on="Sample Channel\nFlow" class="Bool (strict)"("Val(Sgnl)"=w1089) -> ()  [unwired: 2 in, 2 out]
              }
            }
            n686 = node-c288() -> (w1086:T23)  [unwired: 1 in, 3 out]
            n687 = timed-loop "Oscillate AOD" {
              timing: w1086 -> [_]
              timing-out: [_] -> w1085
              tunnel: w1084 -> [w1103]
              tunnel: w1082 -> [w1096]
              i -> [w1105]
              stop <- w1102 stop-if-true
              n688 = node-c288() -> (w1104:i64)  [unwired: 1 out]
              n689 = flat-sequence {
                tunnel: w1105 -> [w1132]
                tunnel: w1104 -> [w1131]
                tunnel: w1103 -> [w1113]
                tunnel: w1096 -> [w1115]
                tunnel: [w1115] -> w1101
                tunnel: [w1114] -> w1100
                tunnel: [w1112] -> w1099
                tunnel: [w1109] -> w1097
                tunnel: w1101 -> [w1177]
                tunnel: w1100 -> [w1175]
                tunnel: w1099 -> [w1174]
                tunnel: [w1173] -> w1098
                tunnel: w1097 -> [w1172]
                tunnel: [w1249] -> w1102
                tunnel: w1098 -> [w1248]
                frame #0 {
                  # "w (rad/s)"
                  # "t (s)"
                  n690 = Divide(x=w1131, y=i64 1000) -> (x/y=w1106:dbl)
                  n691 = local read "BD 1 Frequency 2 (MHz)"() -> (w1108:dbl)
                  n692 = Multiply(x="Osc. freq. (Hz)", y=6.283185307179586) -> (x*y=w1129:dbl)
                  n693 = Multiply(x=w1106, y=w1132) -> (x*y=w1128:dbl)
                  n694 = Multiply(x=w1129, y=w1128) -> (x*y=w1111:dbl)
                  n695 = local read "BD 1 Frequency 1 (MHz)"() -> (w1117:dbl)
                  n696 = case shown="True" w1115 {
                    tunnel: w1111 -> [w1138 w1155]
                    tunnel: w1117 -> [_ w1163]
                    tunnel: w1108 -> [_ w1164]
                    tunnel: [w1135 w1159] -> w1107
                    tunnel: [FALSE w1140] -> w1112
                    tunnel: [0.0 w1151] -> w1109
                    frame False {
                      n697 = Sine(x=w1138) -> (sin(x)=w1136:dbl)
                      n698 = Multiply(x=w1136, y="Osc. amp. (MHz)") -> (x*y=w1135:dbl)
                    }
                    frame True {
                      # "trap position goes from 0 to 1 (0 is when it is furthest away, 1 is when closest)\nso we want to test for tether only when farther away, or x < 1"
                      # "quit if taking too long"
                      # "oscillate the trap"
                      # "Test for tether"
                      n699 = local read "Vec Mean of T1 T2"() -> (w1139:dbl[])
                      "Trigger Signal" <- w1139
                      n700 = Cosine(x=w1155) -> (cos(x)=w1167:dbl)
                      n701 = Subtract(x=w1164, y=w1163) -> (x-y=w1162:dbl)
                      n702 = Decrement(x=w1167) -> (x-1=w1166:dbl)
                      n703 = Subtract(x=w1162, y="Closest Delta (MHz)") -> (x-y=w1160:dbl)
                      n704 = Divide(x=w1166, y=-2.0) -> (x/y=w1150:dbl)
                      n705 = Greater?(x=w1139, y="Stop F (pN)") -> (0:w1157:bool[])
                      n706 = Multiply(x=w1150, y=w1160) -> (x*y=w1159:dbl)
                      n707 = Less?(x=w1150, y="Fish mask thresh") -> (x < y?=w1149:bool)
                      n708 = Boolean To (0,1)(Boolean=w1149) -> (0, 1=w1147:i16)
                      n709 = Multiply(x=w1147, y=w1139) -> (x*y=w1146:dbl[])
                      n710 = Divide(x=w1155, y=6.283185307179586) -> (x/y=w1154:dbl)
                      n711 = Round Toward +Infinity(x=w1154) -> (ceil(x): smallest int >= x=w1151:dbl)
                      "Attempts" <- w1151
                      n712 = Greater?(x=w1146, y="Stop F (pN) (mask)") -> (0:w1144:bool[])
                      n713 = Or Array Elements(Boolean array=w1157) -> (logical OR=w1142:bool)
                      n714 = Or Array Elements(Boolean array=w1144) -> (logical OR=w1141:bool)
                      n715 = Greater?(x=w1151, y="Attempt Limit") -> (0:w1153:bool)
                      n716 = case shown="True" w1153 {
                        frame False {
                        }
                        frame True {
                          n717 = local write "Fish for Tether"(FALSE ("Fish for Tether")) -> ()
                          n718 = call <vilib>:"Beep.vi"() -> ()  [unwired: 3 in, 9 out]
                          n719 = local read "Messages"() -> (w1169:string)
                          n720 = call "Update messages.vi"("Message to add"="Tether fishing timeout." ("Messages"), "Old message string"=w1169) -> ("New message string"=→"Messages":string)
                        }
                      }
                      n721 = Select(t=w1142, s="Normal (on) or masked test (off)", f=w1141) -> (s? t:f=w1140:bool)
                    }
                  }
                  n722 = local read "BD 2 Frequency 1 (MHz)"() -> (w1116:dbl)
                  n723 = Select(t=w1117, s="Scan axis 2", f=w1116) -> (s? t:f=w1120:dbl)
                  n724 = Add(x=w1107, y=w1120) -> (x+y=w1114:dbl)
                  n725 = Select(t=w1114, s="Scan axis 2", f=w1117) -> (s? t:f=w1123:dbl)
                  n726 = Select(t=w1116, s="Scan axis 2", f=w1114) -> (s? t:f=w1122:dbl)
                  n727 = local read "BD 2 Frequency 2 (MHz)"() -> (w1125:dbl)
                  n728 = local read "BD 2 Frequency 3 (MHz)"() -> (w1124:dbl)
                  n729 = local read "Y RF Frequency Limits (MHz)"() -> (w1118:T16)
                  n730 = local read "X RF Frequency Limits (MHz)"() -> (w1119:T16)
                  n731 = local read "BD 1 Frequency 3 (MHz)"() -> (w1126:dbl)
                  n732 = call "set RF board frequency - interlace.vi"("Board 2 Frequency Limits"=w1118, "Board 1 Frequency Limits"=w1119, "FPGA VI Reference In"=w1113, "Board 2 Frequency 3 (MHz)"=w1124, "Board 1 Frequency 3 (MHz)"=w1126, "Board 2 Frequency 2 (MHz)"=w1125, "Board 2 Frequency 1 (MHz)"=w1122, "Board 1 Frequency 2 (MHz)"=w1108, "Board 1 Frequency 1  (MHz)"=w1123) -> ()  [unwired: 1 in, 2 out]
                }
                frame #1 {
                  n733 = And(x=w1177, y=w1174) -> (x .and. y?=w1176:bool)
                  n734 = case "Only if were fishing and now formed tether" shown="True" w1176 {
                    tunnel: w1175 -> [w1179 w1194]
                    tunnel: [w1178 w1193] -> w1173
                    tunnel: w1172 -> [_ w1189]
                    frame False {
                      n735 = local read "Fish for Tether"() -> (w1178:bool)
                      n736 = case shown="False" w1178 {
                        tunnel: w1179 -> [w1180 _]
                        frame False {
                          n737 = property on="BD 1 Frequency 1 (MHz)" class="DigNum (strict)"("Val(Sgnl)"=w1180) -> ()  [unwired: 2 in, 2 out]
                        }
                        frame True {
                        }
                      }
                    }
                    frame True {
                      w1193 = FALSE ("Fish for Tether")
                      n738 = call <vilib>:"Beep.vi"() -> ()  [unwired: 3 in, 9 out]
                      n739 = Number To Decimal String(number=w1189, width (-)=i16 1) -> (decimal integer string=w1187:string)
                      n740 = Concatenate Strings("Formed tether in ", w1187, " attempt(s)." ("string")) -> (w1184:string)
                      n741 = local read "Messages"() -> (w1191:string)
                      n742 = local write "Fish for Tether"(w1193) -> ()
                      n743 = call "Update messages.vi"("Message to add"=w1184, "Old message string"=w1191) -> ("New message string"=w1190:string)
                      n744 = local write "Messages"(w1190) -> ()
                      n745 = Get Date/Time In Seconds() -> (seconds since 1Jan1904=→"Time tether formed":timestamp)
                      n746 = local read "Flow ON during cal?"() -> (w1181:bool)
                      n747 = property on="Sample Channel\nFlow" class="Bool (strict)"("Val(Sgnl)"=w1181) -> (error out=w1182:errorcluster)  [unwired: 2 in, 1 out]
                      n748 = case shown="\"2\", \"3\", \"4\", \"5\", \"6\"" "Then..." {
                        selector: "Then..." -> [_ w1197]
                        tunnel: w1194 -> [w1196 _]
                        tunnel: w1182 -> [_ _]
                        frame "1", Default {
                          n749 = property on="BD 1 Frequency 1 (MHz)" class="DigNum (strict)"("Val(Sgnl)"=w1196) -> ()  [unwired: 2 in, 2 out]
                        }
                        frame "2", "3", "4", "5", "6" {
                          n750 = flat-sequence {
                            tunnel: w1197 -> [w1199]
                            frame #0 {
                              n751 = property on="Trap Delta (MHz)" class="DigNum (strict)"("Val(Sgnl)"="Move to Delta 1 (MHz)") -> ()  [unwired: 2 in, 2 out]
                            }
                            frame #1 {
                              n752 = case shown="\"5\", \"6\"" w1199 {
                                selector: w1199 -> [w1202 w1212 _]
                                frame "3", "4" {
                                n753 = flat-sequence {
                                tunnel: w1202 -> [w1203]
                                tunnel: [w1203] -> w1200
                                tunnel: [w1205] -> w1201
                                tunnel: w1200 -> [w1205]
                                tunnel: w1201 -> [w1209]
                                frame #0 {
                                n754 = property on="Green Laser ON" class="Bool (strict)"("Val(Sgnl)"=TRUE ("Value (Signaling)")) -> ()  [unwired: 2 in, 2 out]
                                }
                                frame #1 {
                                n755 = Multiply(x="Wait Before Save (s)", y=u32 1000 ("x")) -> (x*y=w1207:u32)
                                n756 = Wait (ms)(milliseconds to wait=w1207) -> ()  [unwired: 1 out]
                                }
                                frame #2 {
                                n757 = property on="Start Saving" class="Bool (strict)"("Value"=TRUE ("Start Saving")) -> ()  [unwired: 2 in, 2 out]
                                n758 = case shown="\"4\"" w1209 {
                                frame Default {